vi "UHR-Fleezers Control (host) - Avogadro v1.vi"() -> ()   [LabVIEW 2014]
uses:
  <vilib>/Utility/miscctls.llb/LVPoint32TypeDef.ctl
  <vilib>/Utility/miscctls.llb/LVMinMaxIncTypeDef.ctl
  <vilib>/addons/database/Connection.llb/Conn ObjectReference.ctl
  <vilib>/sound2/lvsound2.llb/Sampling Mode.ctl
  <vilib>/sound2/lvsound2.llb/Sound Data Format.ctl
  <vilib>/Platform/TimedLoop/XDataNode/timing_clust.ctl
  <vilib>/Platform/TimedLoop/XDataNode/nitl_modes.ctl
  <vilib>/Platform/TimedLoop/XDataNode/wakeup.ctl
  <vilib>/userdefined/High Color/nirio_resource_hc.ctl
  uFLUX control_v2/uFLUX control_v2/Pressure Control/Pressure Control.lvclass
  uFLUX control_v2/uFLUX control_v2/TTL/TTL.lvclass
  uFLUX control_v2/uFLUX control_v2/Pressure Control/Pressure Control Config.ctl
  <vilib>/Analysis/baseanly.llb/Mean (DBL).vi
  <vilib>/Instr/_visa.llb/VISA Configure Serial Port (Instr).vi
  <vilib>/FPGAPlugInAG/PCIe-7852R/niLvFpga_Open_PCIe-7852R.vi
  <vilib>/FPGAPlugInAG/PCIe-7852R/niLvFpga_Reset_PCIe-7852R.vi
  <vilib>/Utility/error.llb/Error Cluster From Error Code.vi
  <vilib>/rvi/errors/niLvFpgaAdjustHostInterfaceError.vi
  <vilib>/rvi/interface/common/niFpgaWaitOnOcc.vi
  <vilib>/FPGAPlugInAG/PCIe-7852R/niLvFpga_Run_PCIe-7852R.vi
  <vilib>/express/express analysis/Spectral/Block/exnSpectralBlock spectral measurements PSD poly.vi
  <vilib>/express/express analysis/Spectral/Block/exnSpectralBlock spectral measurements PSD WFM.vi
  <vilib>/Waveform/WDTOps.llb/WDT Append Waveforms DBL.vi
  <vilib>/Waveform/WDTOps.llb/WDT Index Channel DBL.vi
  <vilib>/sound2/lvsound2.llb/Sound Output Write (DBL Single).vi
  <vilib>/FPGAPlugInAG/PCIe-7852R/niLvFpga_Close_PCIe-7852R.vi
  openfpgaref.8.6.ctl
  <vilib>/Platform/TimedLoop/XDataNode/XDataNode.xnode
  <vilib>/rvi/interface/nirviOpenFPGA/nirviOpenFPGA.xnode
  FPGA Bitfiles/UHR-FleezersInst_FPGATarget_UHR-FleezersCont_vcxUwqPIri4.lvbitx
  UHR-Fleezers Control (fpga) - avogadro 2.vi
  <vilib>/rvi/interface/nirviMethod/nirviMethod.xnode
  <vilib>/rvi/interface/nirviReadWriteControl/nirviReadWriteControl.xnode
  <vilib>/express/express analysis/Spectral/XNode/ExpressSpectralMeasurementsBlockNode.xnode
  <vilib>/rvi/interface/nirviCloseFPGA/nirviCloseFPGA.xnode
  <vilib>/Analysis/NI_AALBase.lvlib
  <vilib>/Platform/TimedLoop/XDataNode/XDNodeRunTimeDep.lvlib
  <vilib>/vision/NI_Vision_Development_Module.lvlib
  Duncan Nall/Fluorescence simulation/Global for fluorescence simulation mean (30 samples), (power series).vi
  <vilib>/gmath/NI_Gmath.lvlib
  <vilib>/addons/database/NI_Database_API.lvlib
  <vilib>/rvi/errors/niLvFpgaMergeErrorWithErrorCode.vi
  NiFpgaLv.dll
  <vilib>/FPGAPlugInAG/PCIe-7852R/niLvFpga_ConfigureFifo_PCIe-7852R.vi
  <vilib>/FPGAPlugInAG/PCIe-7852R/niLvFpga_ReadFifo_PCIe-7852R.vi
  <vilib>/addons/database/Connection.llb/DB Tools Open Connec (Path).vi
panel:
  out "APD rates cluster":T1={"APD 1 Rate (Hz)"=4.0, "APD 2 Rate (Hz)"=0.0, "APD 3 Rate (Hz)"=0.0, "Sigma/Mean 1"=nan, "Int Time (s)"=4.0, "Sigma 1"=0.0, "Sigma 2"=0.0, "Sigma 3"=0.0, "Sigma/Mean 2"=nan, "Sigma/Mean 3"=nan}
  in  "Save Event Log?":bool=TRUE
  in  "Bead diameter":dbl=800.0
  in  "Channel 1 Buffer":string
  in  "DNA Construct":string="oligo binding"
  in  "Title":string="testing database"
  in  "Name":string="test name"
  out "Total Time (s) 2":dbl=40.0
  in  "Start Saving":bool
  in  "Comment (data description)":string="testing confocal setup"
  out "Calibrating Trap...":bool
  in  "N sets to save":u32=200 caption="N Sets"
  in  "Save N Sets":bool
  out "Save file name":path=path "C:/Data/180301/180301_027.dat"
  in  "Save ave N":dbl=100.0 caption="Averaging Factor"
  out "Saving...":bool
  in  "Stop Saving":bool
  out "Progress":u16(slide) scale=0.0..100.0
  out "Save Data Rate (Hz)":dbl=1000.0 caption="Rate (Hz)" format="%#_6p"
  out "Save Data Period (s)":dbl=0.001 caption="Period (s)" format="%#_6p"
  in  "Channel 2 Buffer":string="NA"
  in  "Channel 3 Buffer":string="NA"
  out "Read offset current":string(combo)
  out "PSD Y Sum":dbl[](array[numeric])
  out "log file ref":refnum<file>
  out "AL Running":bool
  in  "AL Delay (s)":u32
  in  "Stop assembly line":bool
  in  "Cy5 Fl.  Thresh. (kHz)":dbl=24.5
  in  "Cy3 Fl.  Thresh. (kHz)":dbl=19.0
  in  "Get Fluorophore":bool
  in  "X or Y?":bool=TRUE
  out "Red Fluorophore":bool
  out "Green Fluorophore":bool
  in  "Numeric":dbl
  in  "stop":bool
  in  "Start assembly line":bool
  out "HP3 Flush Time (s)":dbl=90.0
  out "HP1 Flush Time (s)":dbl=60.0
  out "TTrig":cluster{dbl, dbl}(graph)
  in  "Sample Channel\nFlow":bool
  in  "Inject Pump 1":bool
  in  "Inject Pump 3":bool
  in  "Pump 1 contents":string="Bottom: DNA beads" caption="Contents"
  in  "Pump 3 contents":string="Top: ADig beads" caption="Contents"
  out "Time (s)":dbl=32.2
  in  "Index":dbl=27.0 caption="Save File Index" min=1.0 step=1.0
  in  "Scripts":T2(tab)=enum."Cal."
  in  "Experiment position":bool
  in  "Get Bead 1":bool
  in  "Fixed Traps Data\nScript":bool
  in  "Dump spot flow on?":bool=TRUE caption="Flow ON?"
  in  "Daq spot flow on":bool=TRUE caption="Flow ON?"
  in  "Cap 1 Samp Flow ON":bool=TRUE
  in  "Cap 2 Samp Flow ON":bool=TRUE
  in  "Get bead 2":bool
  in  "Get bead 3":bool
  in  "Cap 2 Flow ON":bool=TRUE
  in  "Cap 1 Flow ON":bool=TRUE
  in  "Cap 2 T ON":bool=TRUE
  in  "Move Cap. 2 (ADig Top)":bool
  in  "Move Cap. 1 (DNA Bottom)":bool
  in  "Cal/Data Acq. Spot":bool
  in  "Dump Beads":bool
  in  "Cap 1 T ON":bool=TRUE
  in  "Force FB Data\nScript":bool
  in  "Cap. 2 BD T1?\n(ADig T1, DNA T2)":bool
  in  "Flow Cal":bool
  in  "Pulse Duration (0-100 ms)":dbl=10.0
  in  "Number of pulses For laminar flow":i32=1
  in  "Vent pressure":bool=TRUE
  in  "Pressure Up":bool=TRUE
  in  "Pressure Down":bool=TRUE
  out "Pressure":dbl=0.02073347368347589 format="%#.2f"
  in  "Set zero pressure":bool caption="Vent pressure"
  in  "Vacuum":bool=TRUE
  in  "DAQmx Device Name":tag="Dev1"
  in  "MCL offset scanning range (V)":T3={"Min X"=5, "Max X"=10, "Min Y"=5, "Max Y"=10, "Scan increment"=5.0}
  in  "Multiple-MCL offset?":bool
  in  "Active cal after cal?":bool
  in  "Fish after cal?":bool
  in  "Flow ON during cal?":bool
  in  "Offset 2 Set":dbl=2.0
  in  "Offset 1 Set":dbl
  in  "Cal @ (MHz)":dbl=14.0
  in  "W/ Offset 1":bool=TRUE
  in  "Offset 1 Start (MHz)":dbl=10.0
  in  "W/ Offset 2":bool
  in  "Offset 2 Start (MHz)":dbl=16.0
  in  "Cal Stage Position":i32=3
  in  "Only check fixed trap T2":bool
  in  "Flow ON after\ntether testing?":bool
  in  "Flow ON during \nfishing?":bool
  in  "Fish again after \nraster break?":bool
  in  "Furthest Delta (MHz)":dbl=15.0 step=0.25
  in  "Green ON During Raster":bool
  in  "Move to Delta 2 (MHz)":dbl=12.3
  in  "Attempt Limit":dbl=20.0 caption="Limit"
  out "Attempts":dbl=10.0
  in  "Wait Before Save (s)":u32=1
  in  "Closest Delta (MHz)":dbl=8.0 step=0.25
  in  "Stop F (pN)":dbl=3.0
  in  "Then...":string(combo)="5"
  in  "Move to Delta 1 (MHz)":dbl=10.0
  in  "Tether Alarm?":bool=TRUE
  out "Tether":bool
  in  "TA Cancel Save?":bool
  in  "TA Green Off?":bool
  in  "Raster Set Upon Tether":u32=5
  in  "Save at end (5, 6)":bool
  in  "Stop Fishing When Tether":bool=TRUE
  in  "Delay before dipping (s)":dbl=5.0
  in  "Start dipping after?":bool
  in  "Green ON after FB ON?":bool
  in  "Remove Action Offset":bool
  in  "Stage Position To Establish FB":i32=3
  in  "Trap Trig Fl.":bool
  in  "Starting \nTrap Delta (MHz)":dbl=15.25
  in  "Trap Delta Before Moving":dbl=13.0
  in  "Wait (s)":u32=1
  in  "Green ON":bool
  in  "Start dipping after?":bool=TRUE
  in  "Fixed Traps Trap Delta (MHz)":dbl=15.25 caption="Trap Delta (MHz)"
  out "TTrig Fin Thresh (nm)":dbl
  out "TTrig Sig (nm)":dbl
  out "Threshold stored (nm)":dbl
  in  "Neg. TTrig FPGA":bool=TRUE
  in  "Test ttrig":bool
  in  "Trap Trig. (FPGA)":bool=TRUE
  out "Initializing":bool
  in  "Reinitialize":bool
  out "Triggered":bool
  out "Waiting":bool
  in  "Trap Trig. Fl.":bool
  in  "Wait to get offset (n)":u32=10
  in  "Threshold (nm)":dbl=15.0
  in  "Fl. ON time (n)":i32=90
  out "max value":dbl=-0.9003514563721442
  out "min value":dbl=-1.184251119672945
  in  "Mean T1 Position\nto compare (nm)":dbl caption="Mean T1 for Comparison (nm)" format="%0.2f"
  out "mean":dbl=-1.0423012880225446 format="%0.2f"
  out "standard\ndeviation":dbl=0.2007473770965739 format="%0.2f"
  out "TTrig Sig (Int)":i64
  out "TTrig Fin Thresh (Int)":i64
  in  "FB Trig Integrate":u32=1
  in  "Green ON\nafter start\nreturn?":bool
  in  "Green delay after \nstart return (s)":dbl
  out "Dwell Time (s)":dbl
  in  "FB OFF when \nflow ON":bool
  in  "Flow ON \nduring return\nfrom dip?":bool=TRUE
  in  "Flow ON\nduring daq?":bool=TRUE
  in  "Flow ON\nduring dip?":bool=TRUE
  in  "Cancel dwell":bool
  in  "Pause dwell":bool
  in  "Dwell Duration (s)":i32=45
  in  "Green ON\nbefore dip?":bool
  in  "Cont. Repeat Dipping?":bool=TRUE
  in  "Dipping Delta (MHz)":dbl=15.0
  in  "Move trap \nbefore dip move?":bool
  in  "Save data after return?":bool
  in  "Green ON \nafter return?":bool=TRUE
  in  "Dip Trap Delta 2 (MHz)":dbl=15.0
  in  "Move trap after return?":bool
  in  "Dip Duration (s)":i32=15
  in  "Dip for Protein":bool
  in  "Dip Stage \nPosition":i32=5
  in  "Return Stage \nPosition":i32=3
  out "Dip Time (s)":i32=16
  out "Dip #":i32=5
  in  "Y change (mm)":dbl=-3.0
  in  "Profile":bool
  out "Current Position":cluster{dbl, dbl, dbl}={1.6, 0.50781, -0.0311}
  in  "Shift confocal":bool
  in  "Auto F Reset":bool
  in  "Yank when?":bool
  in  "Yank to which?":bool
  in  "Yank to SP":dbl[](array[numeric])=[-0.128, -0.158, -0.183, -0.21, -0.01, -0.0319, -0.094, -0.143]
  in  "APD to Watch":bool
  out "Duration (s)":dbl=8.399999999999977
  in  "Action":string(combo)="Yank"
  in  "Fl. Triggered...":bool
  in  "Fl. Delta Thresh. (kHz)":dbl=0.14
  out "Waiting":bool
  out "Fl. High":bool
  in  "N pts to average":u16=6
  in  "Yank Delay (s)":dbl=3.0
  in  "Yank to Trap Delta (MHz)":dbl[](array[numeric])=[16.3, 15.85, 14.85]
  in  "N Array El":u8=4 min=1 step=1
  in  "Random Choice":bool=TRUE
  in  "Force Yank":bool
  in  "Reset Force":bool
  in  "N Steps":dbl=20.0
  in  "Step Size (nm)":dbl=0.34
  in  "Save ave factor":dbl=1.0
  in  "Take Stepping Data":bool
  out "Waveform Graph":dbl[](graph) caption="APD Line Scan"
  out "Messages":string="9:07 PM\tUHR-Fleezers ready.\r"
  in  "APD Ave N":dbl=20.0
  in  "Stop All":bool=TRUE
  in  "Tab Control 6":T4(tab)=enum."Display All"
  in  "APD 3 Offset":dbl
  in  "APD 2 Offset":dbl
  in  "APD 1 Offset":dbl
  out "RMS (Ang)":dbl=2.7329016389751146 format="%_2g"
  in  "Bead Sep. Int. Time (s)":dbl=3.0 caption="Int. Time (s)"
  in  "Below (kHz)":dbl=1.0
  in  "Above (kHz)":dbl=2.0
  in  "Adjust Scale\nto Mean":bool
  in  "Remove Offset":bool
  in  "Offset (nm)":dbl format="%#_3g"
  out "Mean":dbl=-361.1793284695809 caption="Mean (pN)" format="%#_3g"
  out "Force":waveform(dbl)[](graph)=[{"t0"=timestamp(302.5999999999914 s since 1904-01-01), "dt"=0.1, "Y"=[-82.15185683561907, -83.09776340587828], "attributes"=variant("NI_ChannelName"=variant(string "T1 X"))}, {"t0"=timestamp(302.5999999999914 s since 1904-01-01), "dt"=0.1, "Y"=[-640.4261792322641, -639.0415144045623], "attributes"=variant("NI_ChannelName"=variant(string "T2 X"))}, {"t0"=timestamp(302.5999999999914 s since 1904-01-01), "dt"=0.1, "Y"=[-361.2890180339416, -361.0696389052203], "attributes"=variant("NI_ChannelName"=variant(string "T1 X"))}]
  out "APD Chart":waveform(dbl)[](graph)=[{"t0"=timestamp(302.5999999999914 s since 1904-01-01), "dt"=0.15, "Y"=[0.0], "attributes"=variant("NI_ChannelName"=variant(string "APD 1"))}, {"t0"=timestamp(302.5999999999914 s since 1904-01-01), "dt"=0.15, "Y"=[0.0], "attributes"=variant("NI_ChannelName"=variant(string "APD 2"))}, {"t0"=timestamp(302.5999999999914 s since 1904-01-01), "dt"=0.15, "Y"=[0.0], "attributes"=variant("NI_ChannelName"=variant(string "APD 3"))}]
  in  "Calibration":u16(ring)=2 items=["None", "Position", "Force"]
  out "T1 X":dbl=-82.62481012074868 caption="T1 X (pN)" format="%0.2f"
  out "T2 X":dbl=639.7338468184132 caption="T2 X (pN)" format="%0.2f"
  out "Bead Separation":waveform(dbl)(graph)={"t0"=timestamp(302.5999999999914 s since 1904-01-01), "dt"=0.1, "Y"=[872.1912647446242, 871.9013680534223], "attributes"=variant("NI_ChannelName"=variant(string "T1 X"))}
  out "Bead Mean (nm)":dbl=872.1413590645118 caption="Mean (nm)" format="%0.2f"
  out "Difference":dbl=557.1090366976646 caption="Difference (pN)" format="%.2g"
  out "Trap Positions":waveform(dbl)[](graph)=[{"t0"=timestamp(302.5999999999914 s since 1904-01-01), "dt"=0.01, "Y"=[3248.000000000121, 3248.000000000121, 3248.000000000121, 3248.000000000121, 3248.000000000121, 3248.000000000121, 3248.000000000121, 3248.000000000121, 3248.000000000121, 3248.000000000121, 3248.000000000121, 3248.000000000121, 3248.000000000121, 3248.000000000121, 3248.000000000121, 3248.000000000121, 3248.000000000121, 3248.000000000121, 3248.000000000121, 3248.000000000121], "attributes"=variant("NI_ChannelName"=variant(string "Trap 1 X"))}, {"t0"=timestamp(302.5999999999914 s since 1904-01-01), "dt"=0.01, "Y"=[6090.0, 6090.0, 6090.0, 6090.0, 6090.0, 6090.0, 6090.0, 6090.0, 6090.0, 6090.0, 6090.0, 6090.0, 6090.0, 6090.0, 6090.0, 6090.0, 6090.0, 6090.0, 6090.0, 6090.0], "attributes"=variant("NI_ChannelName"=variant(string "Trap 2 X"))}, {"t0"=timestamp(302.5999999999914 s since 1904-01-01), "dt"=0.01, "Y"=[2307.4241248817407, 2307.4241248817407, 2307.4241248817407, 2307.4241248817407, 2307.4241248817407, 2307.4241248817407, 2307.4241248817407, 2307.4241248817407, 2307.4241248817407, 2307.4241248817407, 2307.4241248817407, 2307.4241248817407, 2307.4241248817407, 2307.4241248817407, 2307.4241248817407, 2307.4241248817407, 2307.4241248817407, 2307.4241248817407, 2307.4241248817407, 2307.4241248817407], "attributes"=variant("NI_ChannelName"=variant(string "Trap 3 X"))}, {"t0"=timestamp(302.5999999999914 s since 1904-01-01), "dt"=0.01, "Y"=[2608.415338602863, 2608.415338602863, 2608.415338602863, 2608.415338602863, 2608.415338602863, 2608.415338602863, 2608.415338602863, 2608.415338602863, 2608.415338602863, 2608.415338602863, 2608.415338602863, 2608.415338602863, 2608.415338602863, 2608.415338602863, 2608.415338602863, 2608.415338602863, 2608.415338602863, 2608.415338602863, 2608.415338602863, 2608.415338602863], "attributes"=variant("NI_ChannelName"=variant(string "Trap 3 Y"))}]
  in  "Plot Trap Positions":u16(ring)=1 items=["Relative to Base", "Absolute Positions"]
  out "Mean Trap Positions (nm)":T5={"T1 X"=3248.000000000121, "T2 X"=6090.0, "T3 X"=2307.4241248817407, "T3 Y"=2608.415338602863} {"T3 Y" format="%#_6f"; "T3 X" format="%#_6f"; "T2 X" format="%#_6f"; "T1 X" format="%#_6f"}
  out "Trap RMS (ang)":T5
  in  "FB Trap Pos Offset":dbl=-9.744913000168507 caption="Offset (nm)" format="%.1f"
  in  "Rem fb disp offset":bool caption="Rem. Offset"
  in  "Negate Axis":T6
  in  "Trap Pos. Disp. Downsample":dbl=1000.0 caption="Trap Downsample"
  out "Current deltaF (MHz)":dbl=13.999999999999531
  out "Confocal Y 2 (V)":dbl=6.809280068361465
  out "Confocal X 2 (V)":dbl=0.7223435163426621
  out "Confocal Y 1 (V)":dbl=0.7905362102114931
  out "Confocal X 1 (V)":dbl=4.726554155095066
  in  "Set High F Confocal Spot (X-Y)":bool
  in  "Take Detection Laser\nImage":bool
  out "APD 2":T7(plugin-control) caption="APD 2 (Cy5)"
  in  "Flip Green Filter":bool
  in  "Set X Only":bool
  in  "Set Y Only":bool
  out "APD 1":T7(plugin-control) caption="APD 1 (Cy3)"
  out "Detection Laser Y":T7(plugin-control)
  out "Pointer Y (V)":dbl=-0.7646870326853236 format="%_3g"
  out "Pointer X (V)":dbl=3.8578753013702816 format="%_3g"
  in  "Set Confocal Spot (X-Y)":bool
  out "Detection Laser X":T7(plugin-control)
  out "APD 3":T7(plugin-control) caption="APD 3 (Cy2)"
  in  "Display Saved Data":string(combo)
  out "Saved trap pos":dbl[](graph)
  out "Saved APD":dbl[][](graph) caption="Most Recent Time Trace"
  out "Trap Delta Graph":dbl[](graph)=[814.7440815273998, 814.8979753427786, 814.7440815273998, 814.8979753427786, 815.2587973503759, 815.7653893732429, 815.9940245175576, 816.6639538830793, 817.0488179654783, 816.7419405460773, 816.6519036142904, 816.4974989650731, 815.7109069980753, 815.93041988618, 816.1649987450772, 815.809061157495, 815.6741499663872, 815.6132193797599, 815.7326484273603, 815.4258780787427, 815.5285703657568, 815.4105952230886, 815.3637043473332, 815.1766417799918, 815.2066080826977, 815.2952855646151, 815.1577153614937, 815.1483257165202, 815.103698185023, 815.0734640491407, 815.0482295067327, 815.0777239278246, 815.172364970618, 814.8474187596961, 814.7277835545716, 814.9793044780695, 814.6855170853867, 814.412438070411, 814.0439816200725, 813.8468227042506, 814.0504855610436, 814.2421705307053, 814.2890162717929, 814.1656210010467, 814.5529435690976, 814.5856039567557, 814.676050232884, 814.9437232501442, 815.2162112308332, 815.1887960221212, 815.521582230776, 815.6226121996472, 1014.5864122496375, 1009.1265362015508, 992.5482378054153, 986.1956540181214, 972.1584173162003, 965.3728657740866, 949.6805699724813, 943.6828637535813, 926.2066047041824, 919.2501990644666, 900.1260882917104, 891.6687275222423, 871.0999769350776, 862.7496401146702, 839.8232222009757, 830.368999026428, 808.3269081547624, 801.460361191343, 782.8860285419884, 776.888394830104, 761.4006084256285, 757.5035135246504, 748.4316984506299, 742.4168573338349, 734.7495503806092, 731.4190593462148, 723.4184998292208, 719.4308122516741, 707.9353555711359, 703.2416584043925, 693.9776113061731, 688.7511574059804, 678.3621369219416, 673.117062140369, 663.7477524855971, 659.5860627394629, 651.8823950269384, 649.7990028558212, 644.7999959761133, 643.2721744255304, 641.4135306819105, 644.8388324789073, 651.2743025143957, 654.0901369399355, 661.0155952540629, 665.9930553863861, 674.343593063703, 679.6731803348932, 689.7684624678872, 694.683229386238, 704.9146609998086, 708.8471767142431, 718.2964270480468, 721.7635755686134, 731.3138737809775, 734.6764653139262, 740.0494162569726, 746.1952161213528, 755.3485589369287, 759.3529076747604, 775.2360494239853, 780.8947891395995, 795.5815376741821, 802.168356612806, 821.4605678883096, 830.821906026945, 853.367871146864, 861.9665328315244, 883.935149954974, 892.4542343371893, 912.8776488276876, 919.3972144133724, 937.5180585317206, 943.5126129882653, 959.1693940026274, 965.8076864842519, 977.3922231787559, 983.6431060937881, 1002.0572561364202, 1007.5863861915134, 1015.9357376880752, 1009.756590907503, 992.7942478089956, 986.2778615066404, 972.5077549822366, 965.7924234550396, 950.3468484956572, 944.6743090898016, 927.0651990901257, 920.4205432418389, 901.7005066763511, 892.9942632278635, 872.1592253176533, 863.8936831185187, 841.1795233998804, 831.8860760824019, 809.5097476515464, 803.1096243177277, 784.6923861332548, 778.8742440311205, 763.2759096292077, 758.9423709887374, 748.5049803205052, 741.8263228800563, 735.1547242305511, 731.6528136043723, 723.7798739849172, 719.5859985228317, 708.2328909128132, 703.7827595561098, 694.6721065907822, 689.5117553893847, 679.0216738976721, 673.9892076234779, 664.9023163655426, 660.6088839478308, 652.7780873317295, 650.719264076897, 645.7887415701877, 643.603300756574, 641.6488245215564, 645.3579597745344, 651.7485940203541, 654.8342721487169, 661.8514098119371, 666.3790527757451, 674.5346776995054, 679.7494718037921, 687.9903718195691, 692.493130393746, 704.2630686924371, 708.2852457677998, 717.7784376561867, 721.922992460244, 732.3512749580542, 736.5686289087441, 742.6709421593574, 749.0098701359711, 758.1114507061387, 761.7460409773255, 775.1896380879818, 780.4111530407587, 797.0707645360347, 803.3925015317984, 823.000704930262, 832.2034389826387, 855.0712466629764, 863.3490716723319, 885.6239773298603, 894.1467988120052, 914.137511134418, 920.8311115383153, 938.7452548702411, 944.6063307640848, 960.3478831914601, 966.8941350467148, 980.4605904973778, 986.7007819843129, 1000.9846005054333, 1006.5281066537307, 1016.6296759571713, 1010.5613933904026, 991.6315079682045, 984.8972008219537, 972.6023901559429, 965.9794002384867, 950.2609501369502, 944.3726491849254, 924.8400442641083, 918.4390761223503, 901.9985233845349, 893.5385850654884, 872.7883759634178, 863.9910440064057, 841.1621034576366, 831.821915060276, 809.264525120392, 802.8351639028635, 784.4756056802439, 778.3851749761923, 763.1737433274652, 758.5893684422198, 747.5706471457239, 741.0628055306854, 733.1289500382526, 728.8515810712728, 720.6958789988419, 716.8323219477596, 707.7840706735344, 703.1730627771984, 692.7090212226368, 687.4046601176973, 676.7342330802567, 671.4209254227289, 661.8204433684258, 656.6740210818197, 647.9104630636765, 645.1245894630783, 639.6546183765357, 637.433615770073, 635.32185778069, 638.3039462494138, 643.9644675552219, 647.1691751607293, 654.4060401177487, 659.9063595132643, 669.1510079266844, 674.9645963734567, 685.7989607934962, 691.4630742112688, 702.5966563143113, 707.1538430315783, 716.8349303860791, 720.6549113451434, 730.2147114145937, 733.8629940483827, 739.6089872690734, 746.1344965096035, 755.3907183167338, 759.5599925803688, 773.4299518102226, 779.203164570768, 795.7666341776192, 802.1187335097821, 821.4671546262216, 830.6946121590826, 853.5119411586603, 862.1769714359721, 884.2797090908225, 892.7935062989541, 913.0344782134154, 919.7314189473854, 937.5098228501115, 943.3375460030521, 958.7133502961642, 965.0945929750502, 976.4833954545718, 982.9081742047114, 1001.2717725176793, 1007.3700311298576, 1013.6123080257935, 1007.7256952698033, 992.9630905929587, 986.4966228427918, 972.2927572688818, 965.6126534796236, 950.4107290884656, 944.7080625535058, 927.0382944873387, 920.5012477092738, 901.4359347425458, 892.7156639095242, 871.640786733893, 862.868596889059, 839.9676982031876, 830.5388025100877, 808.5163199345462, 801.9197945880541, 784.0502806846813, 778.198261116401, 762.9306964388488, 757.9853995999547, 747.9928221062663, 740.6993579430894, 731.3082702620484, 726.7970637644372, 718.5141940402428, 714.515183453943, 705.9228660684288, 701.6312959858434, 691.830398462303, 687.5034475749161, 677.4085970818354, 672.2498827075515, 662.831292290038, 657.9886368969463, 649.2667395334537, 646.236973677213, 639.7539942696325, 636.0485925204214, 633.7044107935283, 637.6363168361078, 644.5958958378994, 648.3993111481649, 656.6787032353722, 662.3735581116059, 670.9010064057159, 676.3180484713673, 684.4259827619544, 689.140493342598, 699.5791718401742, 704.0134664901375, 717.521268469602, 722.391980431179, 729.7610373779323, 733.2485151277505, 740.0994820931516, 746.4344189451832, 755.0769975529884, 759.1304631987371, 774.6379899257231, 779.9335290298599, 794.5469884363342, 800.9658092241092, 820.9634615010299, 829.9433707158611, 853.1518462047562, 861.6269050773137, 884.0342543779857, 892.3697935543396, 912.5931499999647, 918.661042551916, 936.638926080373, 942.2607601205706, 957.8906911340866, 964.4653309976854, 978.2772182640216, 984.4251980250942, 1000.8002834056629, 1006.2629924981685, 1014.5675560826141, 1009.008002491606, 992.3133825635286, 986.0729465380765, 972.0000087964488, 965.4834793863017, 950.0728418731203, 944.1268181620462, 926.9511252601959, 920.5349539504384, 901.8692375068704, 893.4358884243464, 872.5436472190609, 864.0605270925241, 841.1840174135598, 831.940643047793, 809.122598286512, 802.6871853191689, 784.4687323337431, 778.7927897594092, 763.3837114303572, 758.946488077509, 747.8230796784969, 741.1328138060751, 733.2074430706932, 729.1032127738491, 722.2749951808876, 718.0941302127476, 706.6440092027291, 701.7675913212174, 692.806143733998, 687.8117231771255, 677.1767924694078, 671.8992035654124, 662.3460575383955, 657.7734608562965, 649.8953410441878, 647.5770033821892, 642.2439683694454, 639.8031055547557, 637.7199540606046, 641.7140512723806, 648.0335537535741, 651.2399688149933, 658.6860729414784, 663.6899740791164, 672.3725977835069, 677.5925268427468, 687.6838274828598, 692.693938079121, 703.4685111532244, 708.0516729994206, 719.0336164912973, 722.9100065554113, 731.4168975758136, 735.389965050966, 741.3881376820935, 747.8609192285577, 757.3130158938044, 761.618522484164, 775.5535707108348, 781.2309474479976, 797.5833832537728, 803.3369623135986, 822.2727076054917, 830.8594763452071, 853.4647573059653, 861.6003894977338, 883.7561199748176, 892.2736746877666, 912.5185362678837, 918.8595609471082, 936.8294971701704, 942.6863421236328, 957.9209617708822, 964.4768714866126, 976.2632596722405, 982.485513214422, 1000.7611647478044, 1006.5037001299645, 1014.6935667697063, 1008.6169594208454, 991.7014641449606, 985.1803291447504, 971.2631128238411, 964.6782493546884, 949.2504155873733, 943.5239318827635, 926.119781819186, 919.4064582533576, 900.3900645038808, 891.5033921546526, 870.0588703755352, 861.6387866430484, 839.008139293485, 829.821649735654, 807.7328541243407, 801.4819881204197, 783.5831915981888, 777.9841896434554, 762.7012339570098, 758.5366124555403, 743.7786213422347, 737.1508550256636, 734.2806013304079, 730.6438506778155, 721.5670438329443, 717.8672073953762, 709.1930719055782, 705.1270329795883, 695.0888007382249, 690.777009601925, 680.716354994672, 676.1075419320557, 667.0503153922693, 662.7083188376718, 654.6658738112229, 652.1647459288073, 646.4773120391941, 644.1222416287678, 641.6280177607068, 645.3424692862906, 651.6058295569297, 654.7872231053153, 661.9057540586961, 666.4803413890929, 674.4956560173923, 679.4132317695238, 687.4661398029153, 691.7166894042876, 703.561438996579, 707.7879877508066, 718.8414173479854, 722.8475950807064, 730.1625442469672, 734.0625076406892, 741.2231576804486, 747.7260237346181, 757.0101854335946, 761.0276046110436, 774.7233881611259, 779.8046171432707, 796.0480554501354, 802.2595822627587, 822.1028899340403, 831.7007866975326, 854.8355806328798, 863.4873741819908, 885.485800228946, 893.6047070902878, 913.6628676347256, 919.91941530846, 937.7123406388296, 943.2824057536388, 959.173854967303, 965.5226179786332, 978.9093353436593, 985.0623744822443, 1001.4018238138946, 1006.7937574114176, 1014.85524300114, 1009.171950760574, 990.7150907125415, 984.2533661089808, 972.4191839663073, 966.1229876824639, 951.1022177220403, 945.3071193196581, 928.062205538773, 921.775584041842, 902.8864431279017, 894.3075104654241, 873.4458574688819, 865.1715518015907, 842.5940108800994, 833.4378961104413, 811.4456982166334, 805.2063739299622, 787.1802238328954, 782.0127135891296, 766.7648001664338, 762.7883642066722, 752.1324171459707, 745.6431694264619, 737.455265979983, 733.625015319404, 726.7064582040251, 722.5694326203816, 712.6135186280931, 707.9113691364063, 697.4785489401715, 692.6976927874022, 682.5634170131307, 677.5102837538118, 668.3510667834238, 663.8769644324063, 655.7118134487002, 653.2514211696267, 647.4456972485712, 644.5758808674682, 641.710352581977, 645.212703525538, 650.5037496404831, 653.3419028499911, 660.4508863737387, 665.0267068648866, 672.2199589811593, 677.0114225321269, 686.5630868512438, 690.8574158407605, 702.3980317545386, 707.0391965618388, 717.0490946288515, 720.9939134813399, 729.3418723119967, 733.1068908048962, 741.6131581272982, 748.3626175826614, 756.4802843350857, 761.4531109205958, 775.3203112784082, 781.2614810865476, 798.396544225431, 804.6798129972834, 824.2571691018376, 832.9445484959664, 855.769402465205, 863.7877378543001, 885.9665911047829, 894.3019113309665, 914.5731282962979, 920.8674481389992, 938.6289405723846, 944.168933604735, 959.5355657819257, 965.6443205260973, 976.924994947555, 983.1451542962415, 999.4484481071358, 1005.3004466097797, 1015.959998568259, 1009.8100202297819, 991.1964157036972, 984.4390663905009, 966.8794306745312, 960.2493102382359, 950.7789492317333, 945.0297663191495, 927.8465815578725, 921.518361860597, 902.4004964895094, 893.6174495265539, 872.3590759767035, 863.5316443025641, 840.7121006330547, 831.3885371126936, 809.2935868795372, 803.2250065958697, 784.8895054884767, 779.172966888869, 763.6843692664519, 759.0996908819868, 747.7873075986638, 740.7830950362948, 733.6270094598985, 729.2382767055834, 720.6985527955654, 716.7648546637454, 705.5615222784505, 701.769021147983, 693.7045428282216, 689.2730357469885, 679.3949282695874, 674.6639667785338, 664.2738026384573, 659.549647890286, 650.3549095440853, 647.1445643131949, 642.5715579356373, 639.4243658228568, 637.3823501714388, 641.8248795934013, 649.10881834526, 653.1990811772534, 660.5506047011819, 665.2815924871672, 673.7435908448364, 678.2139882986027, 687.439894610535, 691.682856143945, 700.4164057890008, 704.0228280419041, 716.4671503656854, 720.7966011668002, 729.4485743156215, 734.2126046634569, 740.5258641261654, 747.3732790017518, 756.8518070634259, 761.1415468305345, 774.9363165672144, 780.1093861285556, 797.0247716198162, 803.0268842012232, 822.7558578213878, 831.8953847020575, 854.760421095129, 863.2571176826461, 885.5680782441257, 893.7630636821747, 914.0471129496273, 920.4629586927254, 938.1716229190532, 943.6898042727129, 959.3515949936581, 965.8455535678122, 977.5127593495768, 983.8846724869675, 1002.4348398195118, 1008.043416306873, 1016.3494886221112, 1010.8645293612176, 994.2144901270725, 987.7768180396428, 973.8201562997934, 967.0220473238626, 951.7115972403445, 946.5315192417263, 929.1879748877384, 923.2205732448242, 904.294220421043, 895.7883758035106, 874.6704972289947, 865.6926892051883, 842.5248614820052, 832.8011111480312, 810.2316082218462, 803.1618279870141, 785.0371322961017, 779.0632240730096, 763.5513051465668, 759.1796903417653, 747.9387597197347, 741.9281371030132, 733.7806854358464, 729.1732798036201, 720.6247482323233, 715.9555441808645, 704.2312836393676, 698.9628334745809, 689.8369232635697, 684.7803582369866, 674.1709188030292, 668.4060405800597, 658.9160686896896, 654.1309734988987, 645.5014550108256, 643.0349432456941, 637.0347224683201, 634.4853375203393, 631.9846275404694, 635.5090960068727, 641.5530842819536, 644.660368782498, 652.3651034075214, 657.4473661544962, 666.3778036540677, 671.9938660378823, 682.2171982005144, 687.6733535023725, 698.4766539721137, 703.2430503602296, 713.0990035129422, 717.485427915042, 726.5010493760351, 730.452985856913, 737.7281155918527, 744.3417815368704, 753.7130068899542, 757.7699808868128, 771.5879896219199, 777.0773877916316, 793.9843395919312, 800.0590116545724, 819.8258807310531, 828.9368281733738, 852.164496990814, 860.5944096897033, 882.9362117527382, 891.6626630610307, 911.9787660697525, 918.4064056095086, 936.3109256493376, 941.9664852865745, 957.7390571502976, 963.8398987635753, 977.344135866922, 983.890115449708, 1000.3334019624131, 1006.1324965124392, 1012.7824071270148, 1007.1605883417224, 990.1059218939382, 983.7249504341289, 971.8060806334446, 965.4397922648739, 948.3691262356521, 942.6763099504042, 927.4957399410179, 921.0932844619266, 902.2531622924901, 893.4985973609552, 872.3467351073609, 863.7927613898372, 840.6206208993859, 831.3504198555494, 809.045415022804, 802.7717707857936, 784.5974132436681, 778.8585546701979, 763.1467400198609, 758.3598717146134, 747.0553880349798, 740.1353914168218, 731.4502229308522, 727.1668993297158, 718.938777057816, 714.505582190657, 704.431655796004, 700.4832173153544, 690.5479449289556, 686.2908035709278, 678.1551023207247, 673.2593532615118, 664.7484342992171, 659.9502829700746, 651.5158085161628, 648.077244137653, 641.5605613239868, 637.8093409921313, 635.3639849290258, 639.7760806467898, 645.7809748845729, 650.1066122147386, 656.8975480445478, 662.2969068032548, 670.6416419670046, 675.5555824406804, 685.3160060752307, 689.8027189361878, 699.3398935408211, 703.6681341552644, 716.8079346589378, 721.3742153122915, 730.4111480361242, 734.7398663765671, 741.2257351955182, 748.0352348465997, 757.486188833364, 761.5607260798123, 776.9797427790742, 782.204470441088, 796.9202821029992, 802.3885789507245, 821.7961786218667, 830.5463616039149, 853.4644924245281, 862.0229216776088, 884.4351692759784, 892.7532669864138, 912.6753893970256, 918.9018514220377, 936.7143391608548, 942.2266950661455, 957.7967868646031, 964.2231228754442, 977.7490480480693, 984.4569404001226, 998.892687565973, 1004.5170448855378, 1012.8960430987174, 1006.6903052912606, 991.7538556692546, 984.884843883526, 970.7474776333208, 964.0110102089484, 948.7875865586917, 943.2771033059089, 926.3814943518931, 920.4738254710562, 901.692584505784, 893.3957647367989, 872.4520981302653, 863.7579782180128, 840.7667800681407, 831.1176858767375, 808.5558951677594, 802.0974735077713, 783.8776110474478, 778.2968728651736, 762.9840598894, 758.827037894703, 748.4047210342723, 742.002517401215, 733.8495144130264, 729.6624794336951, 720.9772839764241, 716.4441225623284, 705.5351423649988, 700.6117869988909, 691.1399752967783, 685.342314619424, 675.2982291643737, 670.8023983723702, 660.7296727040574, 656.8128308549478, 650.6474049563751, 648.5924458212502, 642.9496983764263, 640.3931097917514, 638.1519116955061, 641.9059620472875, 648.3839400274643, 651.1581694650384, 658.1203013344868, 661.8195805479382, 669.1015056700841, 674.1432595522913, 684.132228357807, 689.9630222467345, 701.3744835678033, 706.5473748107515, 716.5374469569205, 721.1477978343711, 731.4861364289126, 735.3730305505925, 741.8076665592379, 748.3598760424887, 757.724407270065, 761.6424166821696, 775.4272510628741, 780.9111137502599, 797.5373213111332, 803.6378335115338, 823.0461421759364, 832.0196890089173, 854.9252524639467, 863.0585204844222, 885.2191701011022, 893.3810712712042, 913.2266030153968, 919.5146747914121, 937.0712937182899, 942.2773051526979, 957.4798335897315, 963.9200203400704, 977.4742863135963, 983.7448228825301, 999.980002131369, 1005.7410090779013, 1011.8595293727465, 1006.255619903401, 991.6206615215565, 984.92862510851, 970.9866157071459, 964.3629605632368, 949.0931347825974, 943.5991035900379, 924.2877611227557, 918.0357710771333, 901.2883498561155, 892.7699215310137, 871.8714545986329, 863.3966379153833, 840.7108477441153, 831.7331945720725, 809.5383449481842, 803.6076955277559, 785.8537117447278, 780.7962599365985, 765.5566969903264, 761.932871073352, 751.2102974810857, 744.6904964387637, 736.8590242729066, 733.521301653501, 725.1880116610974, 721.4807032527059, 711.5094305577667, 706.9706357052077, 696.6840976333054, 692.4570130817501, 682.7406071889266, 678.0250036027818, 669.5024248133257, 664.7104293896022, 656.8292162426071, 653.7744202305895, 647.5298033382896, 644.6772955096602, 642.0942230609212, 645.85271459607, 651.2363501618194, 654.3424301838947, 660.6272261199266, 665.1806911120049, 672.8339465365115, 677.3336322489242, 686.5692348367455, 690.5570718482045, 701.0008186420085, 705.6936632368638, 715.4550261973811, 719.8298007725799, 728.972947237091, 733.4793893444867, 742.1096402742003, 748.6773485854819, 756.674196204511, 760.5733079963034, 774.0589759958841, 779.4131830096317, 795.9487859199478, 802.028925700353, 822.0745490824823, 831.2810949242258, 854.6413900390231, 863.0406424121928, 885.8337600367263, 894.2112008163468, 914.2904550166745, 920.5077122500653, 938.1969212475019, 943.6159132216005, 959.1175418848046, 965.4713770338237, 979.1922731397605, 985.8230167235673, 1002.4643547703574, 1008.170358931171, 1014.374095161814, 1008.6674243513428, 993.9583401665715, 987.2228315690369, 972.7090991383409, 966.0068370807184, 948.6306505713975, 942.9565296732662, 927.6504254314079, 921.344162341422, 902.5143168605118, 894.0538627631835, 872.7426449423804, 863.8746717512397, 840.5250409868331, 830.5915156249927, 808.032298838407, 801.6187478448485, 783.2856202135831, 777.9355149753795, 762.6950725277259, 758.6520335198659, 748.0983622844656, 741.7980729990114, 733.7594905645783, 729.371979054234, 722.0114729520795, 717.5761941414698, 705.7292612084664, 701.2168271651415, 692.1628523273122, 687.367972357359, 677.3270744169655, 672.7410429703847, 664.1809601436121, 660.2275767008938, 652.333669269437, 650.1387014709786, 644.6567921538128, 641.692589863572, 639.6088489996133, 643.4483864612447, 649.6134874176475, 652.4023409628714, 659.4610481338589, 663.9003594879126, 671.9054076278811, 676.9906802882327, 686.4653350819033, 691.3020978186505, 702.1564095786746, 707.2756340597371, 717.1600001369808, 721.8182482767468, 731.9949271908285, 735.8709560416881, 741.8901869068562, 747.9502182144771, 758.0372378086637, 762.0135344912122, 774.2329156767344, 779.8410731224262, 796.4988455751778, 802.7857503581132, 822.372806795993, 831.3212216440464, 854.4068976389549, 863.0957032730478, 885.4182305610401, 894.0747171774179, 914.7788133015321, 921.0888386515014, 939.186295364185, 945.066845615798, 960.8827430673698, 967.8337070835958, 981.4629060125424, 988.1034792802043, 1004.3619807669985, 1009.8825886826188, 1018.0652171495727, 1012.2047632226455, 995.3221434816844, 988.616923502088, 972.6021095434767, 965.9276291149035, 952.3424245564665, 946.7840330729517, 929.4028176017384, 922.9068767148573, 903.9755590771226, 895.2815318295524, 874.0178490193365, 864.8239018284927, 841.6574846266165, 831.8787185315999, 808.9079565149576, 802.3633894259184, 783.7505648834903, 777.9061274425904, 762.7794915083476, 758.5259997050952, 747.6348444644433, 741.0565842905784, 733.2200419545945, 728.9216436966209, 720.6184136769858, 716.121409784036, 706.8464334652327, 702.2322959284579, 690.2090765843348, 685.3226280076135, 676.5026328956019, 671.4441386044082, 662.2583772078539, 657.635011797189, 649.1818350041013, 646.1981960098764, 640.1268222930053, 636.8873077224514, 634.4421900522908, 638.0687827571646, 644.5998632124058, 647.8112242827402, 655.3008430549072, 660.1314328252155, 668.3466122375551, 673.458660456955, 682.8504627370419, 687.735875084698, 698.5073405358069, 703.1115660940685, 714.4680286238429, 718.8315376185185, 726.707303993725, 731.2560463314144, 740.0297661290077, 746.8505680436441, 757.0081030104182, 761.1143574259362, 773.464821137015, 778.89490256971, 795.6731299663633, 801.5695061422662, 821.6120248946531, 830.9568664007675, 854.0687743780858, 862.3939909105802, 885.0142162792998, 893.415213189124, 913.4161045160835, 919.6574268942225, 937.3861973012147, 942.855140155199, 958.4912534580928, 965.0284811823833, 978.5889132163157, 984.9597748091545, 999.0972119346595, 1004.4364266488412, 1014.4589569933582, 1008.6656756052216, 989.9668065095657, 983.5756147922666, 971.3386321436602, 964.6604408023314, 949.2937935328271, 943.5187437097757, 926.5290460913878, 920.3415271260162, 901.4845538529758, 893.3237469252367, 872.2776832512776, 863.6911762227676, 840.6408220257448, 830.8713207292828, 808.1603344439256, 801.5399965403797, 783.2635596537905, 777.858416723302, 762.6675932072571, 758.5523499353476, 748.0040064831834, 741.4953546669658, 733.6334154543538, 729.3421318516449, 720.6484543347781, 715.849845660358, 706.2797881326629, 701.1825179136707, 690.8436955631631, 685.7656969471863, 675.6590732001223, 670.8379750631925, 660.7779468078245, 656.9833603062789, 647.7656387968827, 645.7039019139054, 640.7703474290748, 638.5029192004143, 635.788365336397, 638.6914088432704, 644.192745829242, 646.4194000354788, 652.8292601403693, 656.9973434902496, 664.856560537498, 670.1352742340279, 773.8066070205906, 865.6325742299011, 1018.3789731971094, 1017.5324454533746, 1016.821885409221, 1016.2837085807297, 1015.9081950256093, 1015.5619408824314, 1015.535589377951, 1014.8007805780862, 1014.8053089580565, 1014.7513773883505, 1014.5432077879991, 1014.543487131048, 1014.4283434522042, 1014.4448093815607, 1014.5871676326819, 1014.5867241172298, 1014.6461154962675, 1014.8740550642738, 1014.6382432378693, 1014.7696452195694, 1014.9360889414277, 1015.0295406855723, 1015.1072277479507, 1015.0531333167881, 1014.9374450957797, 1014.9004622435352, 1014.7733199178637, 1014.6723796443436, 1014.3327740496081, 1014.4524057610344, 1014.3339793262115, 1014.4091457200389, 1014.5019451488545, 1014.2861643091019, 1014.4945708619964, 1014.3821627961715, 1013.6600685686974, 1013.9756687457639, 1014.0640640192895, 1014.1583313295562, 1014.0724670969782, 1014.0360755501669, 1013.7848057208114, 1013.811591324803, 1013.702497769357, 1014.0662744426907, 1014.0893300083447, 1014.078632283758, 1013.5718613290328, 1013.6901970049049, 1013.7747189744889, 1013.806925687471, 1013.9160752260791, 1013.602757811084, 1013.6100334224407, 1013.3394494499594, 1013.3346196276322, 1013.3241751722006, 1013.4315049236827, 1013.387677533546, 1013.0942370466399, 1013.1380592904891, 1013.074885794508, 1013.0534043022475, 1012.8628771000699, 1012.7242404840446, 1012.6160877167767, 1012.9672613616826, 1013.100643360317, 1013.037299593017, 1013.051812627601, 1013.1666663868286, 1013.3014658850786, 1013.2758911739438, 1013.242746841744, 1013.250094620146, 1013.2333653273112, 1013.3946855823035, 1013.1629542154216, 1013.1996999190953, 1012.7555656347201, 1012.7622630151836, 1012.6967363286454, 1012.680045630929, 1012.8518535105732, 1012.91888063826, 1013.111821408428, 1013.041442728176, 1013.2507724687637, 1012.97910643472, 1013.2890148960915, 1013.1573418977213, 1013.1461505681264, 1013.1524291761243, 1013.1187781007511, 1013.3155542254476, 1013.1997144202799, 1013.2563337148207, 1013.3207049466729, 1013.3966989308412, 1013.3417605115652, 1013.1599919019006, 1013.3285696434352, 1013.1348677716582, 1013.0861306413082, 1013.1242155518573, 1012.9812138712937, 1013.0288004682204, 1013.3758262797727, 1013.2505104991615, 1013.1688031864865, 1013.3386637226071, 1013.4943478269499, 1013.3002172390749, 1013.3292800632951, 1013.5069613821121, 1013.7806715261556, 1014.1155928643634, 1014.4435616086388, 1014.646811925765, 1014.873119910415, 1015.2662304652405, 1014.9154193626514, 1015.1434289104886, 1015.1606745645104, 1015.2375908500587, 1014.9864912757221, 1014.5960701649149, 1014.7386773546452, 1014.5992654858459, 1014.2251009421514, 1013.8038720974546, 1013.572209624798, 1013.5490893678589, 1013.2469421514398, 1013.0204761490107, 1013.4633137184283, 1014.0223790417615, 1013.9425895706022, 1014.3635988090105, 1014.2146139210777, 1014.3130705124862, 1014.4779415677237, 1014.3113891766113, 1014.3665435218803, 1014.2918036182346, 1014.158179765325, 1014.1995245597122, 866.3471030169721, 866.3949598872431, 866.235183760698, 866.3562964172553, 866.2395581741721, 866.4702351038779, 866.5661204001702, 866.388408748011, 866.2789217742595, 866.4533730517326, 866.3165818017544, 866.5607812664068, 866.7718644212191, 866.9397319417579, 867.0113519745885, 867.1432541312874, 867.3261187805703, 867.5454055296614, 867.5244976397641, 867.7496279109639, 867.7600117464632, 868.207087116157, 868.1445329581445, 868.0997249884269, 868.1874320095556, 868.1630616675197, 868.071744529939, 868.1286692882073, 868.019193232964, 868.0714557025591, 868.0259664324194, 867.8544124629858, 867.8663233972508, 867.7029870684847, 867.5116208246642, 867.3809370822224, 867.4841342212849, 867.4471768838972, 867.5418625084505, 867.6018900670101, 867.5934864294982, 867.3356793292804, 867.7984315183483, 867.7203558988692, 867.8970859395502, 868.3008821593364, 868.2272144972608, 868.7227808706559, 868.6684879526094, 868.8658007547682, 1081.20501577867, 1075.2260809914226, 1055.4085959778367, 1048.3328110375587, 1033.3781218648903, 1026.2437871661725, 1012.0174145230254, 1005.7905388471011, 987.7466385489481, 980.9333368851651, 960.5055008631318, 951.8137354860984, 929.7155222546185, 920.7773808784716, 896.4922732112408, 886.7157090048609, 863.1406877658438, 856.2997433671813, 837.1705076810283, 830.8241746539888, 814.5393557072247, 809.7544592527455, 798.0301131861081, 790.8647738557714, 782.4079702847713, 777.8696257820963, 768.7893390436666, 764.1813926400583, 753.1375287005683, 747.9155992203524, 736.8886668440282, 731.7311981649015, 720.9185470697646, 715.6948684354787, 706.0422940761105, 701.1760016428641, 693.7498639955519, 690.5953554994056, 684.3676827606471, 680.9555352244744, 678.1451707857524, 681.7356683042456, 688.3054945778481, 691.7118439154242, 699.3538518827385, 704.7479332226161, 713.6936517130965, 719.3719836280825, 730.1107510623261, 735.7725115382203, 747.7533986291111, 753.1815009235095, 765.2789568473205, 770.0909047979474, 779.8009035650573, 783.9121197426741, 791.8635259701412, 798.6278864757958, 807.0873592465872, 811.5021995242314, 826.3085773663786, 832.1209253720622, 850.0231410866662, 856.7578652113981, 878.1083936242078, 887.7693151247068, 912.513122685548, 921.6077757045618, 945.2806472506524, 953.9950112275802, 974.9858099815586, 981.4371859917283, 1000.1848992128454, 1006.0660191586929, 1022.4476681399836, 1029.4381564648902, 1043.852951098047, 1050.6411094060295, 1067.6738964070742, 1073.2775246285503, 1079.8312592821253, 1074.1942615408605, 1059.2618561526504, 1052.754318262845, 1038.000651741257, 1031.501872389812, 1013.1098313636185, 1007.4264815908, 991.2495547043748, 984.3375377196195, 964.3976903120631, 955.0818480300644, 932.2122631191222, 922.4874259726699, 897.7189288626353, 887.195721208129, 862.8177165503436, 855.5461565969902, 835.4768336907641, 828.9098667577997, 812.2757668610918, 807.4745488943319, 796.488928297203, 789.986745947666, 781.9476606613689, 777.993519069172, 769.2945233540328, 764.6718161575817, 753.0616718489858, 747.2824034940396, 736.0988465579848, 729.5173913089994, 718.026604064719, 712.2032765276172, 703.7593279386845, 699.101073424834, 690.6263208698965, 688.1860191393451, 682.686837936639, 679.9600293176717, 676.779261958434, 680.2664250422041, 686.2449669402824, 689.51326519106, 696.8771659302843, 702.0184951548009, 711.345153535397, 717.7149779923755, 729.0245939407012, 735.3531933548018, 747.9566581871273, 753.8284554288496, 766.2370397033396, 771.2782516543787, 780.4296763391857, 784.1926595441804, 791.7654326451521, 798.6092761647291, 807.1324931623138, 811.6365119197095, 826.6071634074747, 832.8611779532016, 853.2067961228187, 860.1626282239484, 878.8846986882569, 888.6871801824399, 912.610696845145, 920.6772361189478, 944.3349018500952, 953.0769746912364, 974.3225325067447, 980.7921776637044, 999.9074875305611, 1005.3377765230821, 1021.9169478452079, 1028.8097525739206, 1042.9064127330762, 1049.3257992413153, 1066.8809392805028, 1072.8427598186902, 1079.2293040167172, 1072.651860944221, 1054.7086768437093, 1047.5521539692309, 1034.8441029637615, 1027.859818507388, 1009.3766115491247, 1003.5347178255256, 987.306117426452, 980.5133505453523, 960.3136789887305, 951.5246807613535, 929.1095232508262, 920.1936695408655, 895.4471658666828, 885.6488363497954, 861.7973346788422, 854.943928492737, 835.41602461793, 828.9956667392844, 812.7121369138995, 807.7392135651924, 796.155897136892, 789.2053812016136, 780.9992332625411, 776.8932793653435, 768.0018722552737, 763.0979768442312, 751.7807543020607, 746.5474698920837, 734.9839001448909, 729.6598365684747, 718.2566902495995, 712.61669974337, 704.3835479541541, 699.6679219371712, 691.1209007453965, 688.5824841240116, 682.7008974034237, 680.009708464773, 677.1004711056931, 679.3511290830025, 685.0535681368863, 687.6382875147973, 694.8004101150857, 699.3314038978543, 707.5544515645263, 712.905329453944, 722.7931352843697, 728.0100025097801, 739.5961876506111, 744.9820378104263, 756.936647885185, 761.823035694246, 771.4079857501388, 775.9254672973371, 782.691142184669, 789.8737486868579, 801.0866935571555, 805.7630354276928, 820.909596337079, 826.7594840492868, 842.5900588011547, 849.351874687141, 870.4558472328665, 880.516138143346, 904.9479468166573, 913.8148911472312, 937.4655855131672, 946.0725833955694, 967.5633802006361, 974.0321443018985, 993.2133413528034, 999.2834458538066, 1015.9476021986254, 1022.8910573033666, 1037.6702196781366, 1044.6598675520993, 1061.9832240867838, 1067.9853760300653, 1074.81258439275, 1068.7770670459627, 1051.1911941602395, 1044.5192503152361, 1029.818347191804, 1022.6529561605516, 1008.2247533880259, 1002.2256730893824, 983.8691108105132, 977.1803765001721, 957.2395100709044, 948.304980407017, 926.1423239773687, 917.0587257416997, 892.5496086039358, 882.4022103836097, 858.4479929826354, 851.5318398378266, 832.4532848083029, 826.9211278737132, 810.6814365206537, 805.9915000290281, 795.051218636016, 788.5738409346379, 780.2138544075378, 776.1347753148381, 767.6554044509602, 763.0348169358688, 751.5294459929072, 745.9574210701714, 734.2707745002598, 728.4839347887294, 718.886642490458, 713.1705285640486, 701.9832229946023, 697.1683378673893, 690.2632524907827, 688.1316260838225, 682.9755121643287, 680.9739999753925, 678.7081956479785, 681.9278901361611, 687.769594016397, 690.4240441274108, 697.4363785987398, 702.2836678298108, 711.2388024899109, 717.018974339715, 727.9200861702108, 733.7949903088017, 745.5814239313804, 751.0368745765426, 762.7900502373967, 767.0522445215573, 775.4773374021055, 779.39150582122, 786.9160592343974, 793.3860240056842, 803.2582971283214, 807.5040929967166, 820.9253844339336, 826.9195799214135, 845.0296216866973, 851.987929019242, 873.151142089885, 882.6998156133532, 907.029784730483, 915.6082625240341, 939.1420652723816, 947.8745551231816, 969.2580457671437, 975.859990265784, 994.9556132083202, 1001.1083855249719, 1017.6275023897718, 1024.1500071849139, 1038.2997619243656, 1044.9486333194827, 1061.9923483366736, 1067.5376470747692, 1074.1433283491585, 1068.990832397079, 1052.0048695648388, 1045.553980342154, 1033.2198937801409, 1026.9611780550931, 1008.6887401857746, 1002.8020780718351, 986.728781703684, 980.3166209665907, 960.308327899369, 951.7913161724202, 929.5950334913744, 920.9922055604978, 896.9665336001531, 887.3660186991724, 863.3868164497499, 857.1390539202715, 837.857330910781, 832.1315577377944, 816.1430256298756, 811.532737743485, 800.7865969512548, 794.5693298703951, 786.6010530359553, 782.7412440593433, 774.7152353471165, 770.8939303419654, 761.7056505270788, 757.1013436800732, 744.9533272135674, 739.7872110617595, 730.3866777113298, 724.740173344628, 714.4348301278641, 709.2733125846694, 700.0233282245222, 696.7266430753264, 690.2083666420554, 686.8531243677145, 684.0457485236072, 687.5426646923671, 694.0802583841322, 697.5606698051531, 705.5937055212692, 711.0045554907532, 720.6790410766531, 726.7194590181771, 737.551350643621, 743.096174318992, 754.8131612981684, 759.9010195072116, 771.836212397975, 776.4943913184725, 785.5083687427741, 789.8125573771714, 797.8576930392531, 804.7974519785736, 815.0577916989247, 819.3579413874127, 832.3628166188099, 837.65191630736, 855.1966322431812, 861.2954147892076, 881.900516686353, 891.0456662772717, 914.9905426680725, 923.5160180990464, 947.1023642955574, 955.9471928509607, 977.153125446705, 983.6632557356786, 1002.8315989496339, 1008.4304266422898, 1024.9397607546416, 1031.5627795919866, 1045.74221446869, 1052.5886172983978, 1069.8182095076115, 1075.4386057542174, 1082.5468995078472, 1076.7211957564627, 1061.621977956741, 1054.7103170103283, 1039.8425570077693, 1032.8586525055491, 1016.5594163934386, 1010.4717094552419, 991.8576077545424, 985.2014697259738, 964.9346952661759, 956.4998091825009, 935.223677920859, 926.5997765688705, 902.3041793763567, 892.6655913919574, 869.1087568253988, 862.5679606897768, 843.9349217967657, 838.5012634866775, 822.2763188625755, 817.812295315474, 806.5089302348842, 799.9322553083741, 791.8341321840135, 788.022906915609, 779.3830231264793, 774.8744821874171, 763.6765861876987, 758.7007744482278, 747.6055964045825, 742.1637108429081, 732.6103712654633, 727.162177813373, 717.565363608909, 712.8709240997133, 704.2042717780444, 701.9508147591755, 695.8703897026434, 693.1892730642057, 690.2980046560942, 693.6851844195758, 699.3258743291842, 702.5721537027583, 709.4018160104367, 713.9795156014582, 722.950032657215, 728.4912488698344, 739.209048379669, 745.1311534424063, 757.2088024525017, 762.4050585615353, 774.3456181796639, 778.7736558442394, 787.9692569078104, 792.0743947755918, 798.3763643303488, 805.5101037749608, 816.6281464911098, 821.0348333337794, 834.2857802256406, 840.1607620897531, 857.9594668975656, 864.5295329981778, 885.3455149380541, 894.5332390301844, 918.496162154778, 926.7440344799835, 950.2852036797505, 958.809847396674, 979.8752279978467, 986.4973029908754, 1005.2510252288987, 1010.8062321293725, 1027.3407265248293, 1033.935386096155, 1047.9226720929553, 1054.494322149912, 1071.7518526228316, 1077.6882835056385, 873.5897030595041, 873.6176970016281, 873.4215962290258, 873.3486637687383, 873.4865142523765, 873.5475435188766, 874.003086548193, 874.0849252084906, 874.1623495777211, 873.8090158077068, 874.1741997555298, 873.8180472792903, 873.5649594467429, 873.2239226295206, 872.8564858338617, 872.4663390315802, 872.2289919116299, 871.9337813572065, 871.664744697233, 871.5332930057829, 871.4639145053209, 871.3301549740602, 871.3256676329688, 871.1043017924076, 871.0229058634541, 870.9796437221778, 871.2453608652095, 871.027463819015, 871.2582025367797, 871.28577389794, 871.319187774224, 871.4587106178849, 871.3143744778384, 871.4197696743028, 871.3209045694687, 871.2056797607929, 871.5449101997274, 871.2452414961026, 871.2645112965344, 870.9462377466543, 870.3689907231837, 869.6398525982698, 869.534176911412, 870.6289413084746, 871.9395577461198, 872.6968386287384, 872.5409059976955, 872.4856215647457, 872.3620586807026, 871.8099485903347, 1083.9597972940567, 1077.0166331186501, 1056.6629695831352, 1049.4005901766527, 1036.379039340061, 1029.1361726244743, 1010.7068292727246, 1004.3165266972919, 987.9988020109379, 980.7831000509766, 960.7107201978736, 951.4451589602184, 928.5748471789234, 919.2491757549819, 882.0188388376997, 871.8165489508104, 859.876611674847, 852.8089983597474, 833.574919425304, 827.4040345452845, 810.6018096524615, 806.0193604946031, 794.0116082914643, 786.8160721684843, 778.009438446047, 773.8044503116528, 766.7192935377803, 762.0900735629567, 749.8149440364265, 744.7619120624878, 735.320097718786, 729.8876656656129, 718.860381269824, 713.0791733692768, 702.9724581190151, 697.9604622941347, 688.1377749485575, 685.0394627131543, 679.552346267517, 676.6980306525211, 674.4895967144304, 677.977062544897, 684.7525491801075, 688.2398091456178, 696.1308575339023, 701.7195551053321, 710.7353482793128, 716.4971878392357, 726.4760354756002, 732.1397550174613, 743.105926299655, 748.3893111914248, 759.8207482802447, 763.9564849527757, 771.9773079907405, 776.045941248782, 785.7165548471328, 792.09312648095, 801.0304895585493, 805.4015413015441, 820.5323478989853, 826.884324919815, 851.8864741572793, 858.8434835922255, 873.0360542761044, 883.0666766051569, 908.0586600299085, 917.1278817162936, 941.3988986259999, 950.1811240306145, 971.9627643829242, 978.7541618921692, 997.844299416958, 1003.8124449696905, 1020.6641525346345, 1027.4337800232647, 1042.008825874093, 1048.9625311289085, 1066.7199860551368, 1072.768982690544, 1079.386749012788, 1073.0541257280568, 1055.0362966680007, 1047.8968849016728, 1030.9635521442606, 1023.8767087101628, 1011.3964885706818, 1005.1759608865364, 986.7173823451177, 980.0275189385666, 959.6400289335259, 950.6480531607799, 925.1198782304167, 916.7114966017057, 895.1765839437926, 885.1780578671841, 860.9941440139736, 854.0554175904551, 834.0326049801467, 827.119609934663, 810.440524761952, 805.5619385936656, 793.8053412758875, 786.7170781224044, 778.9984121447889, 774.3687351826327, 764.7267629259763, 760.5890024193124, 751.0335024545075, 746.1221949207277, 733.6705575178269, 728.345078768778, 718.7973019356431, 713.0343224933038, 702.9459186452034, 697.1624081170065, 687.7819252047356, 684.0733799478999, 677.4679122553681, 674.5436851667225, 671.8069727916147, 675.3278186566955, 681.9082050809221, 685.909142145931, 694.5026080682995, 700.6452150487637, 710.4586207901458, 716.9810755109901, 728.1074794827, 733.8702140332447, 745.3489089258157, 750.2564711766053, 761.8988451387552, 766.1577934214973, 774.9137058795418, 778.7059065739286, 785.7114481947992, 792.8076100662327, 804.7718258837847, 809.565295871133, 824.9884756483375, 830.8546561550709, 846.3990294797385, 852.9380072531676, 874.1518862698258, 883.7532856977656, 908.3599477311092, 917.51605085256, 941.7137910847333, 950.7390570253506, 972.0120324786436, 978.6522417171954, 997.7972342764376, 